vi "create3Dimg3.vi"(0 "input":u16[][][](array[numeric])=array8x300x2304[5529600 elements], 1 "reverse y":bool, 2 "v comp":dbl=2.0 format="%_4g", 5 "x init pos":dbl[][](array[numeric])=[[-15.0, -15.0, -15.0, -15.0, -15.0, -15.0, -15.0, -15.0], [-15.0, -15.0, -15.0, -15.0, -15.0, -15.0, -15.0, -15.0], [-15.0, -15.0, -15.0, -15.0, -15.0, -15.0, -15.0, -15.0], [-15.0, -15.0, -15.0, -15.0, -15.0, -15.0, -15.0, -15.0], [-15.0, -15.0, -15.0, -15.0, -15.0, -15.0, -15.0, -15.0], [-15.0, -15.0, -15.0, -15.0, -15.0, -15.0, -15.0, -15.0], [-15.0, -15.0, -15.0, -15.0, -15.0, -15.0, -15.0, -15.0], [-15.0, -15.0, -15.0, -15.0, -15.0, -15.0, -15.0, -15.0], [-15.0, -15.0, -15.0, -15.0, -15.0, -15.0, -15.0, -15.0], [-15.0, -15.0, -15.0, -15.0, -15.0, -15.0, -15.0, -15.0], [-15.0, -15.0, -15.0, -15.0, -15.0, -15.0, -15.0, -15.0], [-15.0, -15.0, -15.0, -15.0, -15.0, -15.0, -15.0, -15.0], [-15.0, -15.0, -15.0, -15.0, -15.0, -15.0, -15.0, -15.0], [-15.0, -15.0, -15.0, -15.0, -15.0, -15.0, -15.0, -15.0], [-15.0, -15.0, -15.0, -15.0, -15.0, -15.0, -15.0, -15.0], [-15.0, -15.0, -15.0, -15.0, -15.0, -15.0, -15.0, -15.0]], 7 "correction":T2={"vibration removal"=FALSE, "x correct fast/slow"=TRUE, "y correct fast/slow"=TRUE, "z correct fast/slow"=TRUE}, 9 "AOD scan speed ratio":dbl=5.0, 10 "cropcalib":bool=TRUE, 11 "Nx":dbl=140.25, 12 "reverse x":bool=TRUE, 13 "auto z adjust":T1={"margin"=100.0, "auto z adj"=FALSE, "average"=10, "use given ofst"=FALSE, "given ofst"=10}, 14 "reverse z":bool, 15 "cropcalib data":dbl[][][](array[numeric])=[[[1.2955197191924128, 15.930333155714607, 0.0, 0.2138309419456103], [1.3796957412418465, 38.74653537857694, 0.0, 0.21272660508928573], [1.394661397368111, 41.83536593559279, 0.0, 0.21250095414079084], [1.4008950981088049, 42.449891644190075, 0.0, 0.2124540442621063], [1.3872238827856336, 42.59311909696703, 0.0, 0.2124430158152661], [1.403164903008701, 42.62459302184698, 0.0, 0.21244058752667028], [1.387241055322363, 42.71479003430818, 0.0, 0.21243361901593907], [1.4035837293841666, 42.72079019442731, 0.0, 0.21243315494641554]], [[0.8805634502612065, 137.612759262697, 0.0, 0.1989992782633677], [0.908691333021892, 158.977055996758, 0.0, 0.19480035308532037], [0.9243007848479294, 161.87596871550764, 0.0, 0.1942095651867053], [0.9241322578714062, 162.46966547735272, 0.0, 0.1940880131775804], [0.9126186136828949, 162.63377551685153, 0.0, 0.19405438070036704], [0.9130312609050293, 162.66887951162778, 0.0, 0.19404718468883114], [0.9023552806146711, 162.7658629430556, 0.0, 0.1940273005519781], [0.9116861755350385, 162.80077241635524, 0.0, 0.1940201419831089]], [[0.6818504849580336, 265.7475309200301, 0.0, 0.17115507367984115], [0.6859021068412119, 286.1738895956083, 0.0, 0.16643923244834363], [0.6898328102633684, 288.96429492788536, 0.0, 0.1657952904871067], [0.6985359541050684, 289.5432664146416, 0.0, 0.16566171059368287], [0.701424615082999, 289.7421535644476, 0.0, 0.16561582605687739], [0.6978304304387848, 289.7733541991171, 0.0, 0.16560862799256185], [0.6902138262468043, 289.86802611464844, 0.0, 0.16558678714868522], [0.6904242434107459, 289.9164640000857, 0.0, 0.16557561263047893]], [[0.5770095829784054, 397.86693063682037, 0.0, 0.14129119295257303], [0.5965850174923162, 418.08199088390415, 0.0, 0.13696191712903702], [0.603533152198338, 420.8455092628557, 0.0, 0.13637680938137944], [0.6008854403263229, 421.37756365794536, 0.0, 0.13626434989233094], [0.6032244367757187, 421.6117373389633, 0.0, 0.13621487248532582], [0.5948469125648899, 421.60256903865496, 0.0, 0.1362168093860133], [0.5908906059684114, 421.7282638860769, 0.0, 0.13619025661039585], [0.5975333145376567, 421.7656756426366, 0.0, 0.1361823541187077]], [[0.4351678943725119, 532.7882465994627, 0.0, 0.11415420631385031], [0.44338507561155893, 552.3635454526612, 0.0, 0.11057490688912154], [0.441400120183971, 555.0535806553371, 0.0, 0.11009022307503434], [0.4371961452563937, 555.5938514405896, 0.0, 0.10999308732088403], [0.4601142001999392, 555.9397653049984, 0.0, 0.10993093184259209], [0.44691352537228113, 555.9173506611567, 0.0, 0.10993495854686931], [0.4421388751987365, 556.1138284119112, 0.0, 0.10989966616824481], [0.4386943157048222, 556.072942761175, 0.0, 0.10990700950530265]], [[0.3183847537704878, 670.3578777229392, 0.0, 0.09091612743470276], [0.3341585459230032, 689.668002898644, 0.0, 0.0880037683255728], [0.33358254957482814, 692.3232583149776, 0.0, 0.08760984461542223], [0.3442598833001398, 692.9808829848051, 0.0, 0.08751252541345854], [0.3487775258682859, 693.1792326614213, 0.0, 0.08748319141856081], [0.34539890682748364, 693.1182743270913, 0.0, 0.08749220562990849], [0.33620609482812824, 693.3192893233139, 0.0, 0.08746248368973965], [0.33929497425225463, 693.3819230868993, 0.0, 0.0874532245486372]], [[0.19039663249225214, 810.7140719035333, 0.0, 0.07162477464209875], [0.2003686878989015, 829.5563729147393, 0.0, 0.06936221799574742], [0.19813603021856352, 832.1580991811476, 0.0, 0.06905583979563786], [0.19464784726261541, 832.7211670690875, 0.0, 0.06898972579261202], [0.21215402145503504, 833.0404361667678, 0.0, 0.06895226847626733], [0.20661274045448863, 832.9931638635213, 0.0, 0.06895781317158084], [0.20100778332584923, 833.197816117973, 0.0, 0.06893381244096988], [0.2006853936443349, 833.1907879732481, 0.0, 0.06893463652122724]], [[0.10218618222501163, 954.1070860212964, 0.0, 0.05633656043122527], [0.1097942464293169, 972.6030080519374, 0.0, 0.054688030340087575], [0.10762661885331681, 975.2294142888844, 0.0, 0.05445991856751249], [0.10415952772427772, 975.793187402405, 0.0, 0.054411146702371536], [0.11156707105936903, 976.0550528714073, 0.0, 0.054388516061696125], [0.11676636637696447, 976.1012979701472, 0.0, 0.05438452105387859], [0.10815443372831623, 976.2033688221916, 0.0, 0.054375705016963816], [0.11129737483997815, 976.3501661849938, 0.0, 0.054363029805750106]], [[0.02232193173131236, 1100.458003480752, 0.0, 0.04528679568587693], [0.02944121146475709, 1118.687004530974, 0.0, 0.04422327401618026], [0.02625132591737156, 1121.2407363556383, 0.0, 0.044079607286509614], [0.02112869821831964, 1121.8107009417524, 0.0, 0.04404771979378301], [0.013570277220196658, 1122.0678444115001, 0.0, 0.044033354689010304], [0.023534215593315366, 1122.0580571468322, 0.0, 0.044033901205589976], [0.025747193322899875, 1122.2777764779814, 0.0, 0.04402163676085209], [0.024763124461401276, 1122.369323221604, 0.0, 0.044016529574956845]], [[-0.01851513939925553, 1249.7002645182217, 0.0, 0.03843715621177113], [-0.014642626108013701, 1267.7155887467168, 0.0, 0.0378739458470701], [-0.01801025426925662, 1270.2402713513034, 0.0, 0.03779903171570809], [-0.01742116322026277, 1270.8176889575248, 0.0, 0.0377820342584726], [-0.02212210276957194, 1271.0878687152403, 0.0, 0.03777409831355266], [-0.017477418398414102, 1271.0669079047575, 0.0, 0.0377747135966105], [-0.01811387066510406, 1271.2322711010618, 0.0, 0.037769861336269805], [-0.02126686915426035, 1271.3589501763354, 0.0, 0.03776614698396674]], [[-0.04010248290165919, 1400.654657672175, 0.0, 0.03507915246012616], [-0.03385084696270724, 1418.4250085224824, 0.0, 0.03485222802658161], [-0.0386586680099299, 1420.8074747088365, 0.0, 0.03482384667832894], [-0.038230423749951115, 1421.4050453417635, 0.0, 0.03481680087290129], [-0.04184188155738866, 1421.585789373639, 0.0, 0.03481467548188588], [-0.03825020727276751, 1421.626700264178, 0.0, 0.03481419477365888], [-0.03819421044863702, 1421.835732255688, 0.0, 0.034811740738798225], [-0.03439047238339299, 1421.9873744750103, 0.0, 0.03480996267504943]], [[-0.002241698981151785, 1551.713824633392, 0.0, 0.03380782023383877], [0.0012453405713017673, 1569.2089210631868, 0.0, 0.033726510585873504], [0.004189165947764195, 1571.5849043762348, 0.0, 0.033716050888089155], [0.003353394676480548, 1572.2393892842886, 0.0, 0.03371319233088066], [0.006946375021357198, 1572.4624297787534, 0.0, 0.033712220377738245], [0.006929299396290389, 1572.4767827649644, 0.0, 0.03371215786942128], [0.0018439727972463515, 1572.6103941687347, 0.0, 0.03371157620395815], [-6.589424543790301e-05, 1572.7315853363468, 0.0, 0.033711048955291645]], [[0.10940972578697483, 1700.5036058365686, 0.0, 0.033278462768064454], [0.14030884143215872, 1718.029308276106, 0.0, 0.0332339473396579], [0.1415864150413313, 1720.3287896619054, 0.0, 0.03322841217426742], [0.1400412830763571, 1721.0193785854703, 0.0, 0.033226764694716415], [0.14331232905243496, 1721.1675338176424, 0.0, 0.03322641215808941], [0.13896085196404329, 1721.226857044407, 0.0, 0.03322627108789167], [0.13466760743034456, 1721.4063724875994, 0.0, 0.03322584451513677], [0.13700115410318858, 1721.480103508072, 0.0, 0.03322566944889882]], [[0.30221136926024883, 1845.6462910983516, 0.0, 0.033122027411836896], [0.31038417256991124, 1862.851431090455, 0.0, 0.03315628391697967], [0.309940576407314, 1865.1829197594016, 0.0, 0.033162251652263386], [0.3222153951045925, 1865.8997407956401, 0.0, 0.03316415307774978], [0.33097844860543546, 1866.077449958628, 0.0, 0.03316462934839226], [0.3128481446671003, 1866.1468213355697, 0.0, 0.03316481579524222], [0.3121891912197725, 1866.2899532037077, 0.0, 0.03316520142246926], [0.3196247412383286, 1866.3605366714753, 0.0, 0.03316539205414948]], [[0.6456214667424263, 1984.7072942331238, 0.0, 0.0340201109036844], [0.6678939026910484, 2001.664525334681, 0.0, 0.034244514470616494], [0.6786392099097327, 2003.9259338299069, 0.0, 0.03427649195036153], [0.6694953411343931, 2004.5602304339345, 0.0, 0.03428554727712729], [0.6740182914502384, 2004.7101934506484, 0.0, 0.03428769367564932], [0.6777530059790706, 2004.8210396530947, 0.0, 0.034289281552464246], [0.6673923387494938, 2004.8690703617433, 0.0, 0.03428996995118894], [0.6763830703022506, 2005.0174353744337, 0.0, 0.034292097750119765]], [[1.2236158728431121, 2115.0099485030305, 0.0, 0.036329787536892866], [1.23685071458803, 2131.486241347703, 0.0, 0.036673232133765055], [1.246468607832611, 2133.6181978902264, 0.0, 0.03671712639323843], [1.2546462321518845, 2134.2850123031512, 0.0, 0.036730816493420804], [1.2548195165125549, 2134.4096350599025, 0.0, 0.036733372914504514], [1.2795018086993082, 2134.6262324019913, 0.0, 0.03673781438918411], [1.2598791365136606, 2134.6378644631554, 0.0, 0.03673805285292886], [1.2569232666415076, 2134.7038364538093, 0.0, 0.0367394052002723]]]) -> (4 "zyx":u16[][][](array[numeric]), 8 "z ofst":dbl)   [LabVIEW 2024]
uses:
  <vilib>/Analysis/baseanly.llb/Mean (DBL).vi
  Global variables/global for picoscope.vi
  <vilib>/gmath/NI_Gmath.lvlib
  <vilib>/Analysis/NI_AALBase.lvlib
panel:
  out "Waveform Graph":dbl[](graph)=[1115.9, 1124.8, 1133.0, 1145.4, 1170.8, 1175.1999999999998, 1153.4, 1128.8, 1093.8, 1062.9, 1035.8000000000002, 1012.1, 991.1, 962.0, 910.2, 869.5, 837.3, 800.4, 760.0999999999999, 730.9, 703.2, 681.5999999999999, 659.5, 637.0, 615.7, 601.0, 589.5, 576.2, 565.7, 551.4, 537.0, 514.1, 497.3, 488.0, 483.2, 471.5, 453.8, 436.4, 417.4, 393.7, 370.29999999999995, 354.2, 342.7, 329.4, 317.2, 308.6, 301.3, 297.2, 297.4, 299.8, 300.70000000000005, 300.70000000000005, 298.8, 298.5, 299.70000000000005, 300.70000000000005, 302.0, 305.29999999999995, 307.5, 308.79999999999995, 311.3, 315.6, 319.4, 324.5, 327.4, 330.8, 336.4, 340.4, 347.79999999999995, 355.3, 365.0, 373.9, 388.7, 403.4, 420.1, 440.3, 455.79999999999995, 473.3, 494.4, 516.3, 533.5, 551.4, 568.8, 583.4, 595.1, 604.7, 619.4, 633.4000000000001, 641.5999999999999, 652.5, 681.9000000000001, 717.7, 707.3, 728.9555555555555, 744.775, 762.6285714285714, 779.0666666666666, 795.4, 817.55, 837.3333333333333]
  out "Waveform Graph 3":u16[](graph)=[609, 625, 732, 595, 485, 479, 415, 411, 460, 467, 497, 576, 587, 552, 532, 506, 428, 382, 369, 377, 405, 409, 414, 467, 507, 526, 453, 370, 327, 373, 405, 363, 358, 381, 374, 308, 281, 280, 277, 251, 225, 197, 164, 138, 140, 142, 153, 146, 144, 146, 138, 139, 139, 137, 144, 147, 138, 141, 139, 147, 141, 149, 145, 150, 143, 145, 149, 158, 158, 165, 169, 171, 168, 157, 181, 181, 169, 170, 176, 185, 181, 207, 217, 217, 202, 232, 270, 258, 264, 326, 319, 303, 326, 360, 388, 396, 401, 481, 399, 429, 426, 444, 499, 457, 439, 449, 452, 448, 402, 487, 515, 494, 478, 499, 529, 533, 532, 495, 571, 661, 627, 594, 598, 501, 449, 437, 420, 442, 438, 438, 505, 498, 578, 589, 553, 534, 536, 530, 522, 575, 528, 503, 480, 552, 592, 630, 622, 671, 728, 664, 610, 627, 734, 596, 486, 433, 417, 405, 410, 400, 387, 365, 307, 279, 256, 231, 187, 198, 158, 164, 141, 152, 136, 136, 141, 144, 138, 141, 147, 153, 145, 149, 138, 141, 144, 136, 142, 147, 147, 158, 158, 150, 149, 160, 158, 153, 169, 172, 152, 153, 154, 152, 166, 169, 168, 176, 185, 172, 178, 198, 181, 186, 176, 185, 196, 194, 236, 240, 237, 251, 309, 321, 325, 367, 339, 333, 398, 399, 388, 379, 382, 379, 354, 322, 348, 377, 371, 365, 496, 573, 147]
  out "Array 2":dbl[][](array[numeric])
  out "Array":dbl[][](array[numeric])
  out "Numeric 3":i32=8
  in  "discrete(T)/seq(F)":bool
  out "Numeric 2":i32=16
  out "Numeric":i32=300
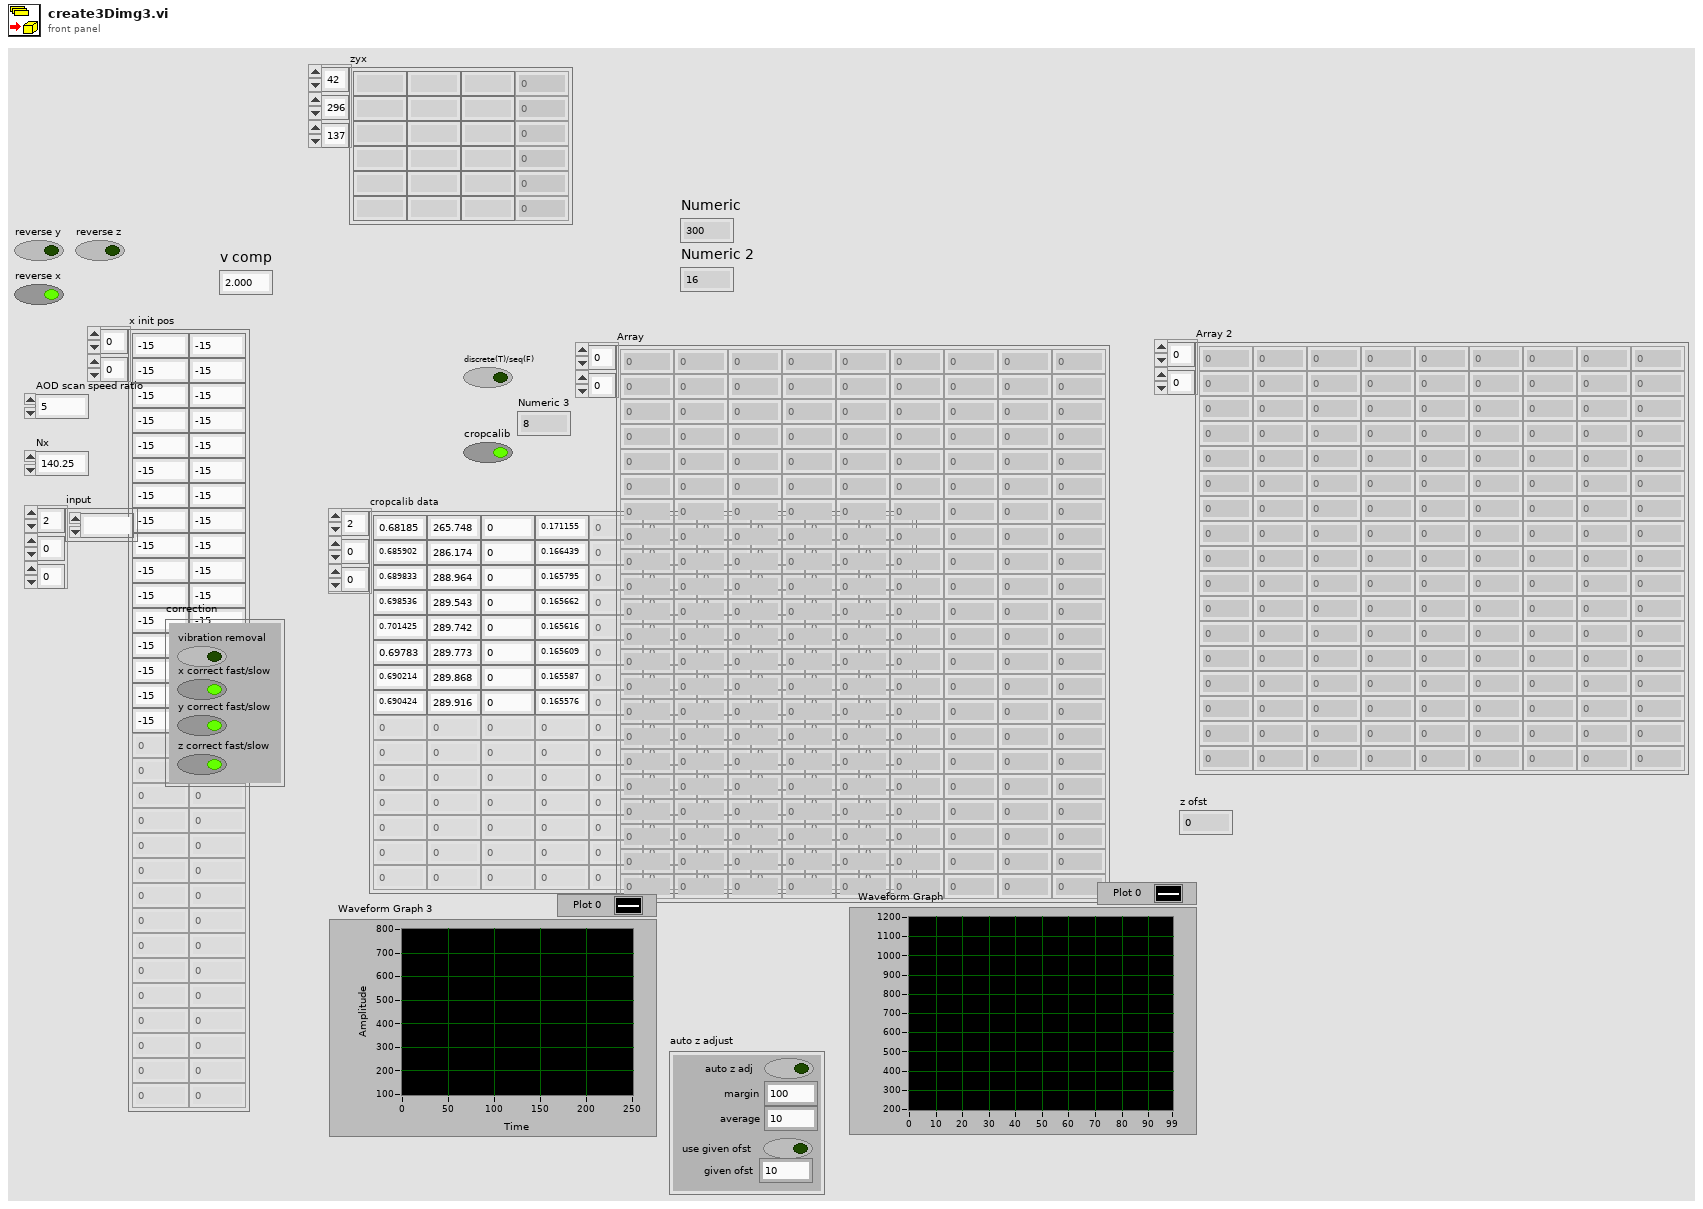
[diagram p1: front panel]
types:
  T1 = cluster{"margin":dbl, "auto z adj":bool, "average":i32, "use given ofst":bool, "given ofst":i32}
  T2 = cluster{"vibration removal":bool, "x correct fast/slow":bool, "y correct fast/slow":bool, "z correct fast/slow":bool}
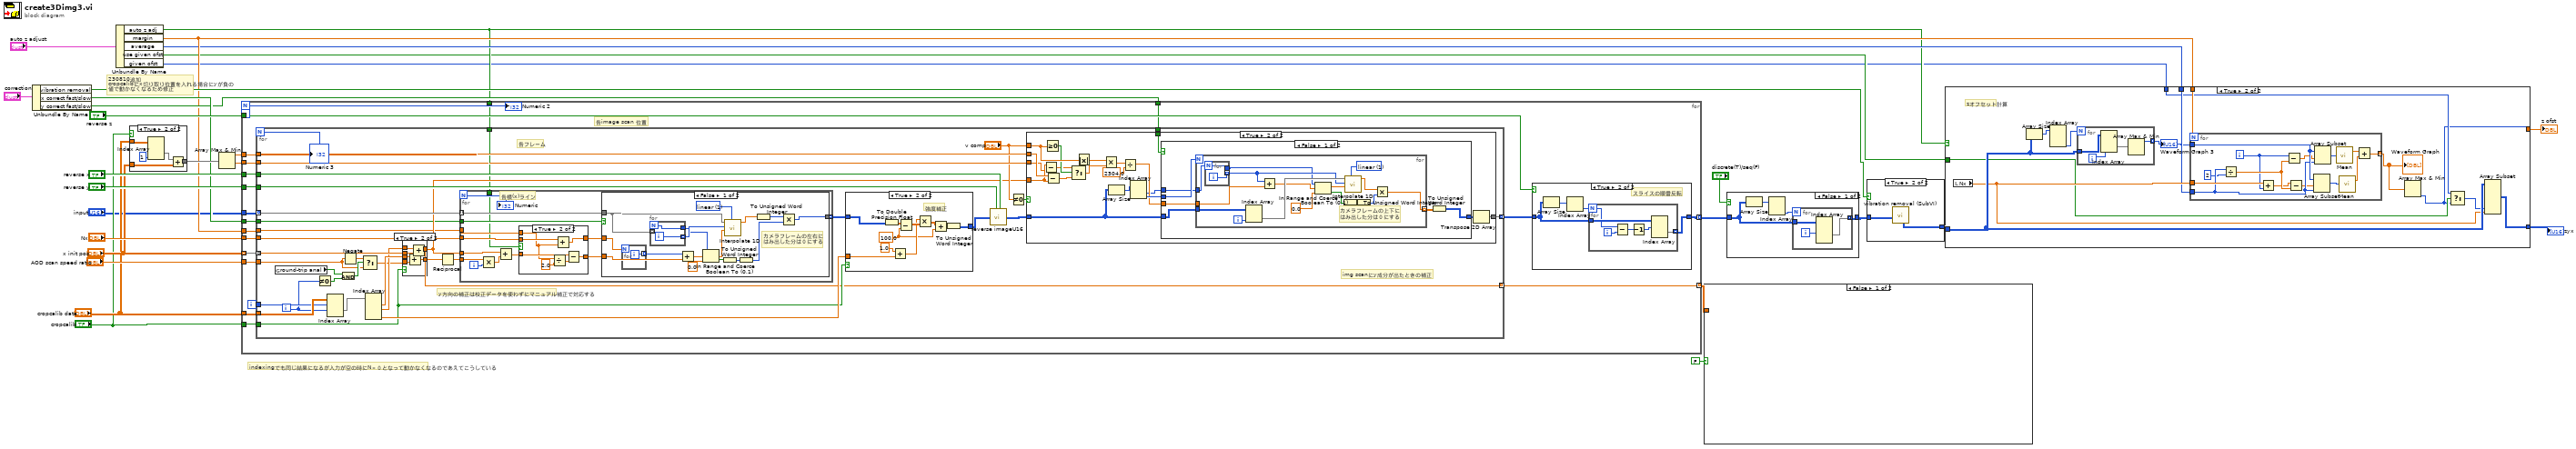
[diagram p0: block diagram]
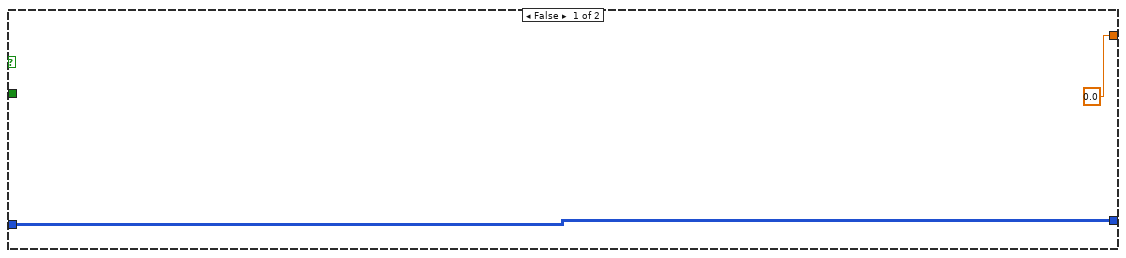
[diagram p2: hidden frame]
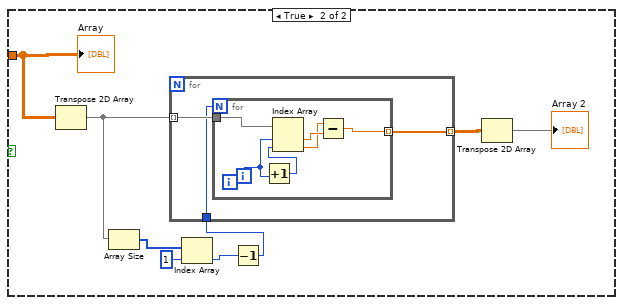
[diagram p5: hidden frame]
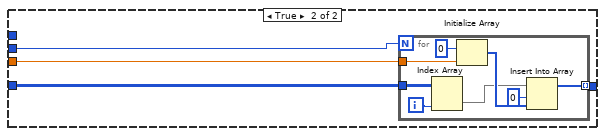
[diagram p11: hidden frame]
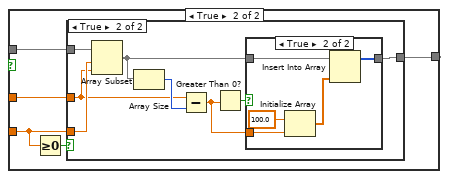
[diagram p13: hidden frame]
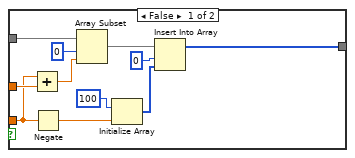
[diagram p14: hidden frame]
diagram:
  # "230810追加\ncropcalibにx切り取り位置を入れる場合にyが負の値で動かなくなるため修正"
  # "indexingでも同じ結果になるが入力が空の時にN＝０となって動かなくなるのであえてこうしている"
  n1 = Unbundle By Name("correction") -> ("vibration removal"=w12:bool, "x correct fast/slow"=w13:bool, "y correct fast/slow"=w11:bool)
  n2 = Unbundle By Name("auto z adjust") -> ("auto z adj"=w4:bool, "margin"=w7:dbl, "average"=w6:i32, "use given ofst"=w3:bool, "given ofst"=w2:i32)
  n3 = case shown="True" "cropcalib" {
    tunnel: "x init pos" -> [w31 w36]
    tunnel: [w31 w34] -> w18
    tunnel: "cropcalib data" -> [_ w33]
    frame False {
    }
    frame True {
      n4 = Index Array(array=w33, index (dim 2)=1 ("disabled index (col)")) -> (element=w32:dbl[][])  [unwired: 2 in]
      n5 = Add(x=w32, y=w36) -> (x+y=w34:dbl[][])
    }
  }
  n6 = Array Max & Min(array=w18) -> (max value=w24:dbl, min value=w23:dbl)  [unwired: 2 out]
  n7 = for {
    N -> [w51]
    tunnel: "x init pos" -> [w56] mode=indexing
    tunnel: "Nx" -> [w42]
    tunnel: "AOD scan speed ratio" -> [w48]
    tunnel: "input" -> [w55]
    tunnel: "reverse x" -> [w54]
    tunnel: "reverse y" -> [w53]
    tunnel: "reverse z" -> [w52]
    tunnel: w24 -> [w50]
    tunnel: w23 -> [w49]
    tunnel: "cropcalib data" -> [w47]
    tunnel: "cropcalib" -> [w46]
    tunnel: [w44] -> w22 mode=indexing
    tunnel: [w43] -> w20 mode=indexing
    tunnel: w13 -> [w41]
    tunnel: w11 -> [w40]
    tunnel: w7 -> [w39]
    tunnel: w4 -> [w38]
    workers-P: _ -> [_]
    i -> [w45]
    # "各image scan 位置"
    n8 = for {
      N -> [w81]
      tunnel: w55 -> [w91] mode=indexing
      tunnel: [w97] -> w37 mode=indexing
      tunnel: w48 -> [w68]
      tunnel: w42 -> [w101]
      tunnel: w56 -> [w95] mode=indexing
      tunnel: w54 -> [w99]
      tunnel: w53 -> [w100]
      tunnel: w50 -> [w96]
      tunnel: w49 -> [w94]
      tunnel: w47 -> [w83]
      tunnel: w46 -> [w84]
      tunnel: w45 -> [w82]
      tunnel: [w80] -> w43 mode=indexing
      tunnel: w41 -> [w78]
      tunnel: w40 -> [w77]
      tunnel: w39 -> [w76]
      tunnel: w38 -> [w75]
      i -> [w74]
      # "img scanにy成分が出たときの補正"
      # "y方向の補正は校正データを使わずにマニュアル補正で対応する"
      # "各フレーム"
      n9 = global read "global for picoscope.vi" "round-trip anal"() -> (w73:bool)
      n10 = Not Equal To 0?(x=w74) -> (x != 0?=w72:bool)
      n11 = Index Array(array=w83, index (dim 0)=w82, index (dim 1)=w74) -> (element=w79:dbl[])  [unwired: 1 in]
      n12 = And(x=w73, y=w72) -> (x .and. y?=w71:bool)
      n13 = Negate(x=w68) -> (-x=w70:dbl)
      n14 = Select(t=w70, s=w71, f=w68) -> (s? t:f=w69:dbl)
      n15 = Index Array(array=w79) -> (element #1=w89:dbl, element #2=w88:dbl, element #4=w86:dbl)  [unwired: 4 in, 1 out]
      n16 = case shown="True" w84 {
        tunnel: w69 -> [w114 w121]
        tunnel: w95 -> [w115 w120]
        tunnel: [w115 w119] -> w80
        tunnel: [w114 w118] -> w90
        tunnel: w89 -> [_ w117]
        tunnel: w88 -> [_ w116]
        frame False {
        }
        frame True {
          n17 = Add(x=w117, y=w121) -> (x+y=w118:dbl)
          n18 = Add(x=w116, y=w120) -> (x+y=w119:dbl)
        }
      }
      n19 = Reciprocal(x=w90) -> (1/x=w102:dbl)
      n20 = for {
        N -> [w185]
        tunnel: w91 -> [w191] mode=indexing
        tunnel: w80 -> [w190]
        tunnel: w102 -> [w187]
        tunnel: [w186] -> w87 mode=indexing
        tunnel: w101 -> [w183]
        tunnel: w78 -> [w184]
        tunnel: w76 -> [w179]
        tunnel: w75 -> [w178]
        i -> [w189]
        # "各横(x)ライン"
        n21 = Multiply(x=w187, y=w189) -> (x*y=w188:dbl)
        n22 = Add(x=w190, y=w188) -> (x+y=w180:dbl)
        n23 = case shown="True" w178 {
          tunnel: w183 -> [w193 w200]
          tunnel: [w193 w199] -> w182
          tunnel: [w192 w198] -> w181
          tunnel: w180 -> [w192 w195]
          tunnel: w179 -> [_ w194]
          frame False {
          }
          frame True {
            n24 = Divide(x=w194, y=2.0) -> (x/y=w196:dbl)
            n25 = Add(x=w200, y=w194) -> (x+y=w199:dbl)
            n26 = Subtract(x=w195, y=w196) -> (x-y=w198:dbl)
          }
        }
        n27 = case shown="False" w184 {
          tunnel: w191 -> [w215 w224]
          tunnel: [w201 w223] -> w186
          tunnel: w182 -> [w214 w222]
          tunnel: w181 -> [w212 w220]
          frame False {
            w209 = 1 items=["nearest", "linear", "spline", "cubic Hermite", "Lagrange"] ("method")
            # "カメラフレームの左右に\nはみ出した分は０にする"
            n28 = for {
              N: w214 -> [_]
              tunnel: [w217] -> w213 mode=indexing
              i -> [w217]
            }
            n29 = for {
              N -> [w218]
              tunnel: w215 -> [_] mode=indexing
              tunnel: [w219] -> w216 mode=indexing
              tunnel: [w218] -> w207
              i -> [w219]
            }
            n30 = Add(x=w213, y=w212) -> (x+y=w211:dbl[])
            n31 = In Range and Coerce(upper limit=w207, x=w211, lower limit=0.0) -> (coerced(x)=w208:dbl[], In Range?=w205:bool[])
            n32 = Boolean To (0,1)(Boolean=w205) -> (0, 1=w204:i16[])
            n33 = call <vilib>:"Interpolate 1D.vi"("method"=w209, "xi"=w208, "X"=w216, "Y"=w215) -> ("yi"=w210:dbl[])  [unwired: 5 in, 2 out]
            n34 = To Unsigned Word Integer(number=w204) -> (unsigned 16bit integer=w203:u16[])
            n35 = To Unsigned Word Integer(number=w210) -> (unsigned 16bit integer=w202:u16[])
            n36 = Multiply(x=w202, y=w203) -> (x*y=w201:u16[])
          }
          frame True {
            n37 = Greater Or Equal To 0?(x=w220) -> (x >= 0?=w221:bool)
            n38 = case shown="True" w221 {
              tunnel: w224 -> [w235 w243]
              tunnel: [w225 w238] -> w223
              tunnel: w220 -> [w231 w242]
              tunnel: w222 -> [w233 w236]
              frame False {
                n39 = Add(x=w231, y=w233) -> (x+y=w232:dbl)
                n40 = Negate(x=w231) -> (-x=w230:dbl)
                n41 = Array Subset(array=w235, index=0, length=w232) -> (w226:u16[])
                n42 = Initialize Array(u16 100 ("element"), w230) -> (w228:u16[])
                n43 = Insert Into Array(array=w226, index=0, new element=w228) -> (w225:u16[])
              }
              frame True {
                n44 = Array Subset(array=w243, index=w242, length=w236) -> (w237:u16[])
                n45 = Array Size(array=w237) -> (size(s)=w241:i32)
                n46 = Subtract(x=w236, y=w241) -> (x-y=w239:dbl)
                n47 = Greater Than 0?(x=w239) -> (x > 0?=w240:bool)
                n48 = case shown="True" w240 {
                  tunnel: w237 -> [w244 w249]
                  tunnel: w239 -> [_ w248]
                  tunnel: [w244 w245] -> w238
                  frame False {
                  }
                  frame True {
                    n49 = Initialize Array(100.0 ("element"), w248) -> (w246:dbl[])
                    n50 = Insert Into Array(array=w249, new element=w246) -> (w245:u16[])  [unwired: 1 in]
                  }
                }
              }
            }
          }
        }
        "Numeric" <- w185
      }
      n51 = case shown="True" w84 {
        tunnel: w87 -> [w103 w104]
        tunnel: w86 -> [_ w109]
        tunnel: [w103 w105] -> w85
        frame False {
        }
        frame True {
          w107 = 100.0
          # "強度補正"
          n52 = To Double Precision Float(number=w104) -> (double precision float=w112:dbl[][])
          n53 = Add(x=1.0 ("element"), y=w109) -> (x+y=w110:dbl)
          n54 = Subtract(x=w112, y=w107) -> (x-y=w113:dbl[][])
          n55 = Multiply(x=w110, y=w113) -> (x*y=w108:dbl[][])
          n56 = Add(x=w108, y=w107) -> (x+y=w106:dbl[][])
          n57 = To Unsigned Word Integer(number=w106) -> (unsigned 16bit integer=w105:u16[][])
        }
      }
      n58 = call "reverse imageU16.vi"("output array in"=w85, "reverse v"=w100, "reverse h"=w99) -> ("output array out"=w98:u16[][])
      n59 = Not Equal To 0?(x="v comp") -> (x != 0?=w93:bool)
      n60 = case shown="True" w93 {
        tunnel: w98 -> [w122 w139]
        tunnel: [w122 w137] -> w97
        tunnel: w96 -> [_ w134]
        tunnel: w80 -> [_ w133]
        tunnel: w94 -> [_ w132]
        tunnel: "v comp" -> [_ w131]
        tunnel: w77 -> [_ w123]
        frame False {
        }
        frame True {
          n61 = Subtract(x=w133, y=w132) -> (x-y=w129:dbl)
          n62 = Greater Or Equal To 0?(x=w131) -> (x >= 0?=w130:bool)
          n63 = Subtract(x=w134, y=w133) -> (x-y=w128:dbl)
          n64 = Select(t=w129, s=w130, f=w128) -> (s? t:f=w127:dbl)
          n65 = Absolute Value(x=w131) -> (abs(x)=w126:dbl)
          n66 = Multiply(x=w126, y=w127) -> (x*y=w136:dbl)
          n67 = Array Size(array=w139) -> (size(s)=w141:i32[])
          n68 = Divide(x=w136, y=2304.0) -> (x/y=w125:dbl)
          n69 = Index Array(array=w141) -> (element #1=w124:i32, element #2=w140:i32)  [unwired: 2 in]
          n70 = case shown="False" w123 {
            tunnel: w140 -> [w145 w169]
            tunnel: w139 -> [w147 w168]
            tunnel: [w142 w167] -> w138
            tunnel: w125 -> [w146 w166]
            tunnel: w124 -> [w144 _]
            frame False {
              n71 = for {
                N: w145 -> [_]
                tunnel: w147 -> [w163]
                tunnel: [w151] -> w143 mode=indexing
                tunnel: w146 -> [w156]
                tunnel: w144 -> [w161]
                i -> [w162]
                w160 = 1 items=["nearest", "linear", "spline", "cubic Hermite", "Lagrange"] ("method")
                # "カメラフレームの上下に\nはみ出した分は０にする"
                n72 = for {
                  N: w161 -> [w164]
                  tunnel: [w165] -> w158 mode=indexing
                  tunnel: [w164] -> w153
                  i -> [w165]
                }
                n73 = Index Array(array=w163, index (col)=w162) -> (element=w159:u16[])  [unwired: 1 in]
                n74 = Add(x=w158, y=w156) -> (x+y=w157:dbl[])
                n75 = In Range and Coerce(upper limit=w153, x=w157, lower limit=0.0) -> (coerced(x)=w155:dbl[], In Range?=w149:bool[])
                n76 = Boolean To (0,1)(Boolean=w149) -> (0, 1=w152:i16[])
                n77 = call <vilib>:"Interpolate 1D.vi"("method"=w160, "xi"=w155, "X"=w158, "Y"=w159) -> ("yi"=w148:dbl[])  [unwired: 5 in, 2 out]
                n78 = To Unsigned Word Integer(number=w152) -> (unsigned 16bit integer=w150:u16[])
                n79 = Multiply(x=w148, y=w150) -> (x*y=w151:dbl[])
              }
              n80 = To Unsigned Word Integer(number=w143) -> (unsigned 16bit integer=w142:u16[][])
            }
            frame True {
              n81 = for {
                N: w169 -> [_]
                tunnel: w168 -> [w177]
                tunnel: [w173] -> w167 mode=indexing
                tunnel: w166 -> [w170]
                i -> [w176]
                n82 = Index Array(array=w177, index (col)=w176) -> (element=w172:u16[])  [unwired: 1 in]
                n83 = Initialize Array(u16 0 ("element"), w170) -> (w174:u16[])
                n84 = Insert Into Array(array=w172, index=0 ("f"), new element=w174) -> (w173:u16[])
              }
            }
          }
          n85 = Transpose 2D Array(2D array=w138) -> (transposed array=w137:u16[][])
        }
      }
      "Numeric 3" <- w81
    }
    n86 = case shown="True" w52 {
      tunnel: w37 -> [w57 w59]
      tunnel: [w57 w58] -> w44
      frame False {
      }
      frame True {
        # "スライスの順番反転"
        n87 = Array Size(array=w59) -> (size(s)=w61:i32[])
        n88 = Index Array(array=w61) -> (element=w60:i32)  [unwired: 1 in]
        n89 = for {
          N: w60 -> [w65]
          tunnel: w59 -> [w67]
          tunnel: [w62] -> w58 mode=indexing
          i -> [w66]
          n90 = Subtract(x=w65, y=w66) -> (x-y=w64:i32)
          n91 = Decrement(x=w64) -> (x-1=w63:i32)
          n92 = Index Array(array=w67, index (dim 0)=w63) -> (element=w62:u16[][])  [unwired: 2 in]
        }
      }
    }
    "Numeric 2" <- w51
  }
  n93 = case shown="False" FALSE {
    tunnel: w20 -> [_ w257]
    frame False {
    }
    frame True {
      n94 = Transpose 2D Array(2D array=w257) -> (transposed array=w256:dbl[][])
      n95 = Array Size(array=w256) -> (size(s)=w255:i32[])
      n96 = Index Array(array=w255, index=1) -> (element=w253:i32)
      n97 = Decrement(x=w253) -> (x-1=w251:i32)
      n98 = for {
        tunnel: w256 -> [w260] mode=indexing
        tunnel: [w259] -> w252 mode=indexing
        tunnel: w251 -> [w258]
        n99 = for {
          N: w258 -> [_]
          tunnel: w260 -> [w265]
          tunnel: [w262] -> w259 mode=indexing
          i -> [w261]
          n100 = Increment(x=w261) -> (x+1=w264:i32)
          n101 = Index Array(array=w265, index #1=w261, index #2=w264) -> (element #1=w266:dbl, element #2=w263:dbl)
          n102 = Subtract(x=w263, y=w266) -> (x-y=w262:dbl)
        }
      }
      n103 = Transpose 2D Array(2D array=w252) -> (transposed array=→"Array 2":dbl[][])
      "Array" <- w257
    }
  }
  n104 = case shown="False" "discrete(T)/seq(F)" {
    tunnel: w22 -> [w268 w275]
    tunnel: [w267 w274] -> w15
    frame False {
      n105 = Array Size(array=w268) -> (size(s)=w270:i32[])
      n106 = Index Array(array=w270) -> (element #2=w269:i32)  [unwired: 2 in, 1 out]
      n107 = for {
        N: w269 -> [_]
        tunnel: w268 -> [w273]
        tunnel: [w271] -> w267 mode=concatenating
        i -> [w272]
        n108 = Index Array(array=w273, index (dim 1)=w272) -> (element=w271:u16[][][])  [unwired: 3 in]
      }
    }
    frame True {
      n109 = for {
        tunnel: w275 -> [w276] mode=indexing
        tunnel: [w276] -> w274 mode=concatenating
      }
    }
  }
  n110 = case shown="True" w12 {
    tunnel: w15 -> [w277 w279]
    tunnel: [w277 w278] -> w10
    frame False {
    }
    frame True {
      n111 = call "vibration removal (SubVI).vi"("Array in"=w279) -> ("Array out"=w278:u16[][][])  [unwired: 6 in, 4 out]
    }
  }
  n112 = case shown="True" w4 {
    tunnel: w10 -> [w281 w294]
    tunnel: [w281 w293] -> w9
    tunnel: w7 -> [_ w291]
    tunnel: w6 -> [_ w290]
    tunnel: [0.0 w282] -> w5
    tunnel: w2 -> [_ w284]
    tunnel: w3 -> [_ w285]
    frame False {
    }
    frame True {
      # "zオフセット計算"
      n113 = local read "Nx"() -> (w292:dbl)
      n114 = Array Size(array=w294) -> (size(s)=w289:i32[])
      n115 = Index Array(array=w289) -> (element #3=w288:i32)  [unwired: 3 in, 2 out]
      n116 = for {
        N: w288 -> [_]
        tunnel: w294 -> [w312]
        tunnel: [w309] -> w287 mode=indexing
        i -> [w311]
        n117 = Index Array(array=w312, index (dim 2)=w311) -> (element=w310:u16[][])  [unwired: 2 in]
        n118 = Array Max & Min(array=w310) -> (max value=w309:u16)  [unwired: 3 out]
      }
      "Waveform Graph 3" <- w287
      n119 = for {
        N: w291 -> [_]
        tunnel: w290 -> [w301]
        tunnel: w287 -> [w308]
        tunnel: w292 -> [w307]
        tunnel: [w302] -> w286 mode=indexing
        i -> [w298]
        n120 = Divide(x=w301, y=2) -> (x/y=w299:dbl)
        n121 = Add(x=w307, y=w298) -> (x+y=w297:dbl)
        n122 = Subtract(x=w298, y=w299) -> (x-y=w296:dbl)
        n123 = Subtract(x=w297, y=w299) -> (x-y=w295:dbl)
        n124 = Array Subset(array=w308, index=w295, length=w301) -> (w305:u16[])
        n125 = Array Subset(array=w308, index=w296, length=w301) -> (w306:u16[])
        n126 = call-poly <vilib>:"Mean.vi"("X"=w306) -> ("mean"=w304:dbl)  [unwired: 1 out]
        n127 = call-poly <vilib>:"Mean.vi"("X"=w305) -> ("mean"=w303:dbl)  [unwired: 1 out]
        n128 = Add(x=w304, y=w303) -> (x+y=w302:dbl)
      }
      "Waveform Graph" <- w286
      n129 = Array Max & Min(array=w286) -> (min index (indices)=w282:i32)  [unwired: 3 out]
      n130 = Select(t=w284, s=w285, f=w282) -> (s? t:f=w283:i32)
      n131 = Array Subset(array=w294, index (dim 2)=w283, length (dim 2)=w292) -> (w293:u16[][][])  [unwired: 4 in]
    }
  }
  "zyx" <- w9
  "z ofst" <- w5
